vi "Trajectory Builder.vi"() -> ()   [LabVIEW 2025]
uses:
  Types/Limits.ctl
  Types/Overrides.ctl
  Types/Trajectory Data.ctl
  Types/Segment Type.ctl
  Types/Path Type.ctl
  Types/Drive Type.ctl
  Types/Angluar Limits.ctl
  Types/Command Editor Info.ctl
  Types/Single Cmd Info.ctl
  <vilib>/picture/picture.llb/imagedata.ctl
  <vilib>/Utility/miscctls.llb/LVPositionTypeDef.ctl
  <vilib>/Utility/miscctls.llb/LVRowAndColumnTypeDef.ctl
  Types/Internal Path Stuff.ctl
  <vilib>/event_ctls.llb/lveventtype.ctl
  6a65ebb4-e776-4ba2-b94f-6ff829af6114.vi
  6a65ebb4-e776-4ba2-b94f-6ff829af6114.vi/c0db33a9-eb6c-44d9-b982-8563e05d2734.vi
  6a65ebb4-e776-4ba2-b94f-6ff829af6114.vi/ae3535a8-0066-4e8d-a5de-b07ac05a7c65.vi
  6a65ebb4-e776-4ba2-b94f-6ff829af6114.vi/dda8e586-731b-4197-ad83-6a4d05585a0a.vi
  Global Settings.vi
  <vilib>/Utility/cursorutil.llb/Set Cursor (Icon Pict).vi
  <vilib>/Comparison/Less/Less Functor/Less Functor.lvclass
panel:
  in  "Correct at Beginning \nof Path":bool
  in  "Zero Translational\n Velocity":bool
  in  "Pickup Balls":bool
  in  "Delete":bool
  out "Picture":picture
  in  "New Page Selector":T1(radio)
  in  "Push":bool
  out "?":bool
  out "RS":bool=TRUE
  in  "Cache":T5
  in  "Zero Velocity":bool
  in  "Reverse Path":bool
  in  "Robot Backwards":bool
  out "Duration (s)":dbl format="%#.4g"
  out "Distance (ft)":dbl format="%#.1g"
  in  "Instructions":string="Directions:\nUse mouse to ...\n    move robot position (rectangle with arrow)\n    rotate robot (red arrow)\n    move waypoints (numbered circles)\nClick in open space to add a waypoint\nShift click to delete a waypoint\nHover over a waypoint and use arrow keys to nudge\n\nTime slider and Play button will run robot along path to test for collisions.\n\nNew creates a new path at default location\n\nAppend creates a path using current path's position and heading.\n\nTo add a command, move robot using Time slider and double click the Command in Palette.\n\nYou can modify command timing in the graph or Command Sequencer tree.\n\nEnable/disable a command by clicking on the enable column item.\n\nDelete a command by shift-clicking in the enable column.\n\nTo configure command parameters, Select the command name in the tree, Open Panel, enter parameters, and Inhale the parameters.\n\nYou may sometimes want to type values into WayPoints directly.\n\nOverrides allow you to set accel and V limits for any turn."
  out "Command Palette":picture
  in  "Directory":bool
  in  "Tab Control":T1(tab)
  in  "Vertical Reflection":bool
  in  "Angular Limits":T6={"Velocity (deg/s)"=6.0, "Accel (deg/s^2)"=360.0, "Jerk (deg/s^3)"=1000.0} {"Jerk (deg/s^3)" min=0.01 step=1.0; "Accel (deg/s^2)" min=0.01; "Velocity (deg/s)" min=0.01}
  in  "Path Type":T7
  in  "Overrides":T8=[{"Count"="1", "Angular Override"=0.0, "Enabled?"=FALSE, "Velocity Override"=6.0, "Angle Override"=nan}] {"Angle Override" step=5.0; "Velocity Override" step=5.0; "Angular Override" step=5.0}
  in  "Horizontal Reflection":bool
  in  "Sample Period (s)":dbl=0.02 min=0.001 max=1.0 format="%#_6p"
  in  "Limits":T9={"Velocity (fps)"=6.0, "Accel (fps^2)"=15.0, "Jerk (fps^3)"=150.0, "StoopidFast (fps)"=6.0} {"StoopidFast (fps)" min=0.01; "Jerk (fps^3)" min=0.01 step=1.0; "Accel (fps^2)" min=0.01; "Velocity (fps)" min=0.01}
  in  "Conditions":T10 {"vFinal (fps)" min=0.0; "vInitial (fps)" min=0.0}
  in  "Drive Type":T11=enum."Holonomic"
  in  "Turn Rate (Bezier)":dbl=5.0 format="%#_13g"
  in  "Origin Reflection":bool
  in  "Current Limit":dbl=50.0 min=0.01
  in  "WayPoints":cluster{"x":dbl, "y":dbl, "th":dbl}[](array[cluster])
  in  "Turn Angle Limit (deg)":dbl=90.0
  in  "Allow Angles > 90":bool=TRUE
  in  "Stoopid Overlap %":dbl min=0.0
  in  "Unjank":bool
  in  "Turn Deceleration":bool=TRUE
  in  "Turn Acceleration":bool=TRUE
  out "Trajectory Data":T12
  in  "Open Command":bool
  in  "Inhale":bool
  in  "Command Sequence":string(tree)
  in  "Projects":u16(ring) items=["Rebuilt 2468.lvproj"]
  in  "Refresh":bool
  in  "Snap to foot":bool
  in  "Angle Limiter":enum16{"90", "45", "15", "1"}(ring)=enum."15"
  in  "Snap robot to baseline":bool
  in  "Background":u16(ring) items=["Rebuilt", "Reefscape"]
  in  "Robot Color":u32(colorbox)=14421504
  out "Field Size (ft)":cluster{"width":dbl, "height":dbl}={"width"=26.4166, "height"=57.5729} {"width" format="%#.2g"; "height" format="%#.2g"}
  in  "Robot Size (in)":cluster{"width":dbl, "height":dbl}={"width"=24.0, "height"=30.0}
  in  "Hide Path":bool
  in  "Time (s)":dbl(slide) scale=0.0..1.6400000000000001 scale format="%#.1g"
  in  "Play":bool
  out "fps":dbl[](graph)
  in  "Append":bool
  in  "Open":i32[](listbox)
  in  "Filename":string
  in  "Save":bool
  in  "New":bool
  # "Command Palette"
  # "StupidFast makes each linear segment into a\nvelocity ramp to max speed (for clothoid paths only)"
  # "Nicotine"
  # "A"
  # "V"
  # "O"
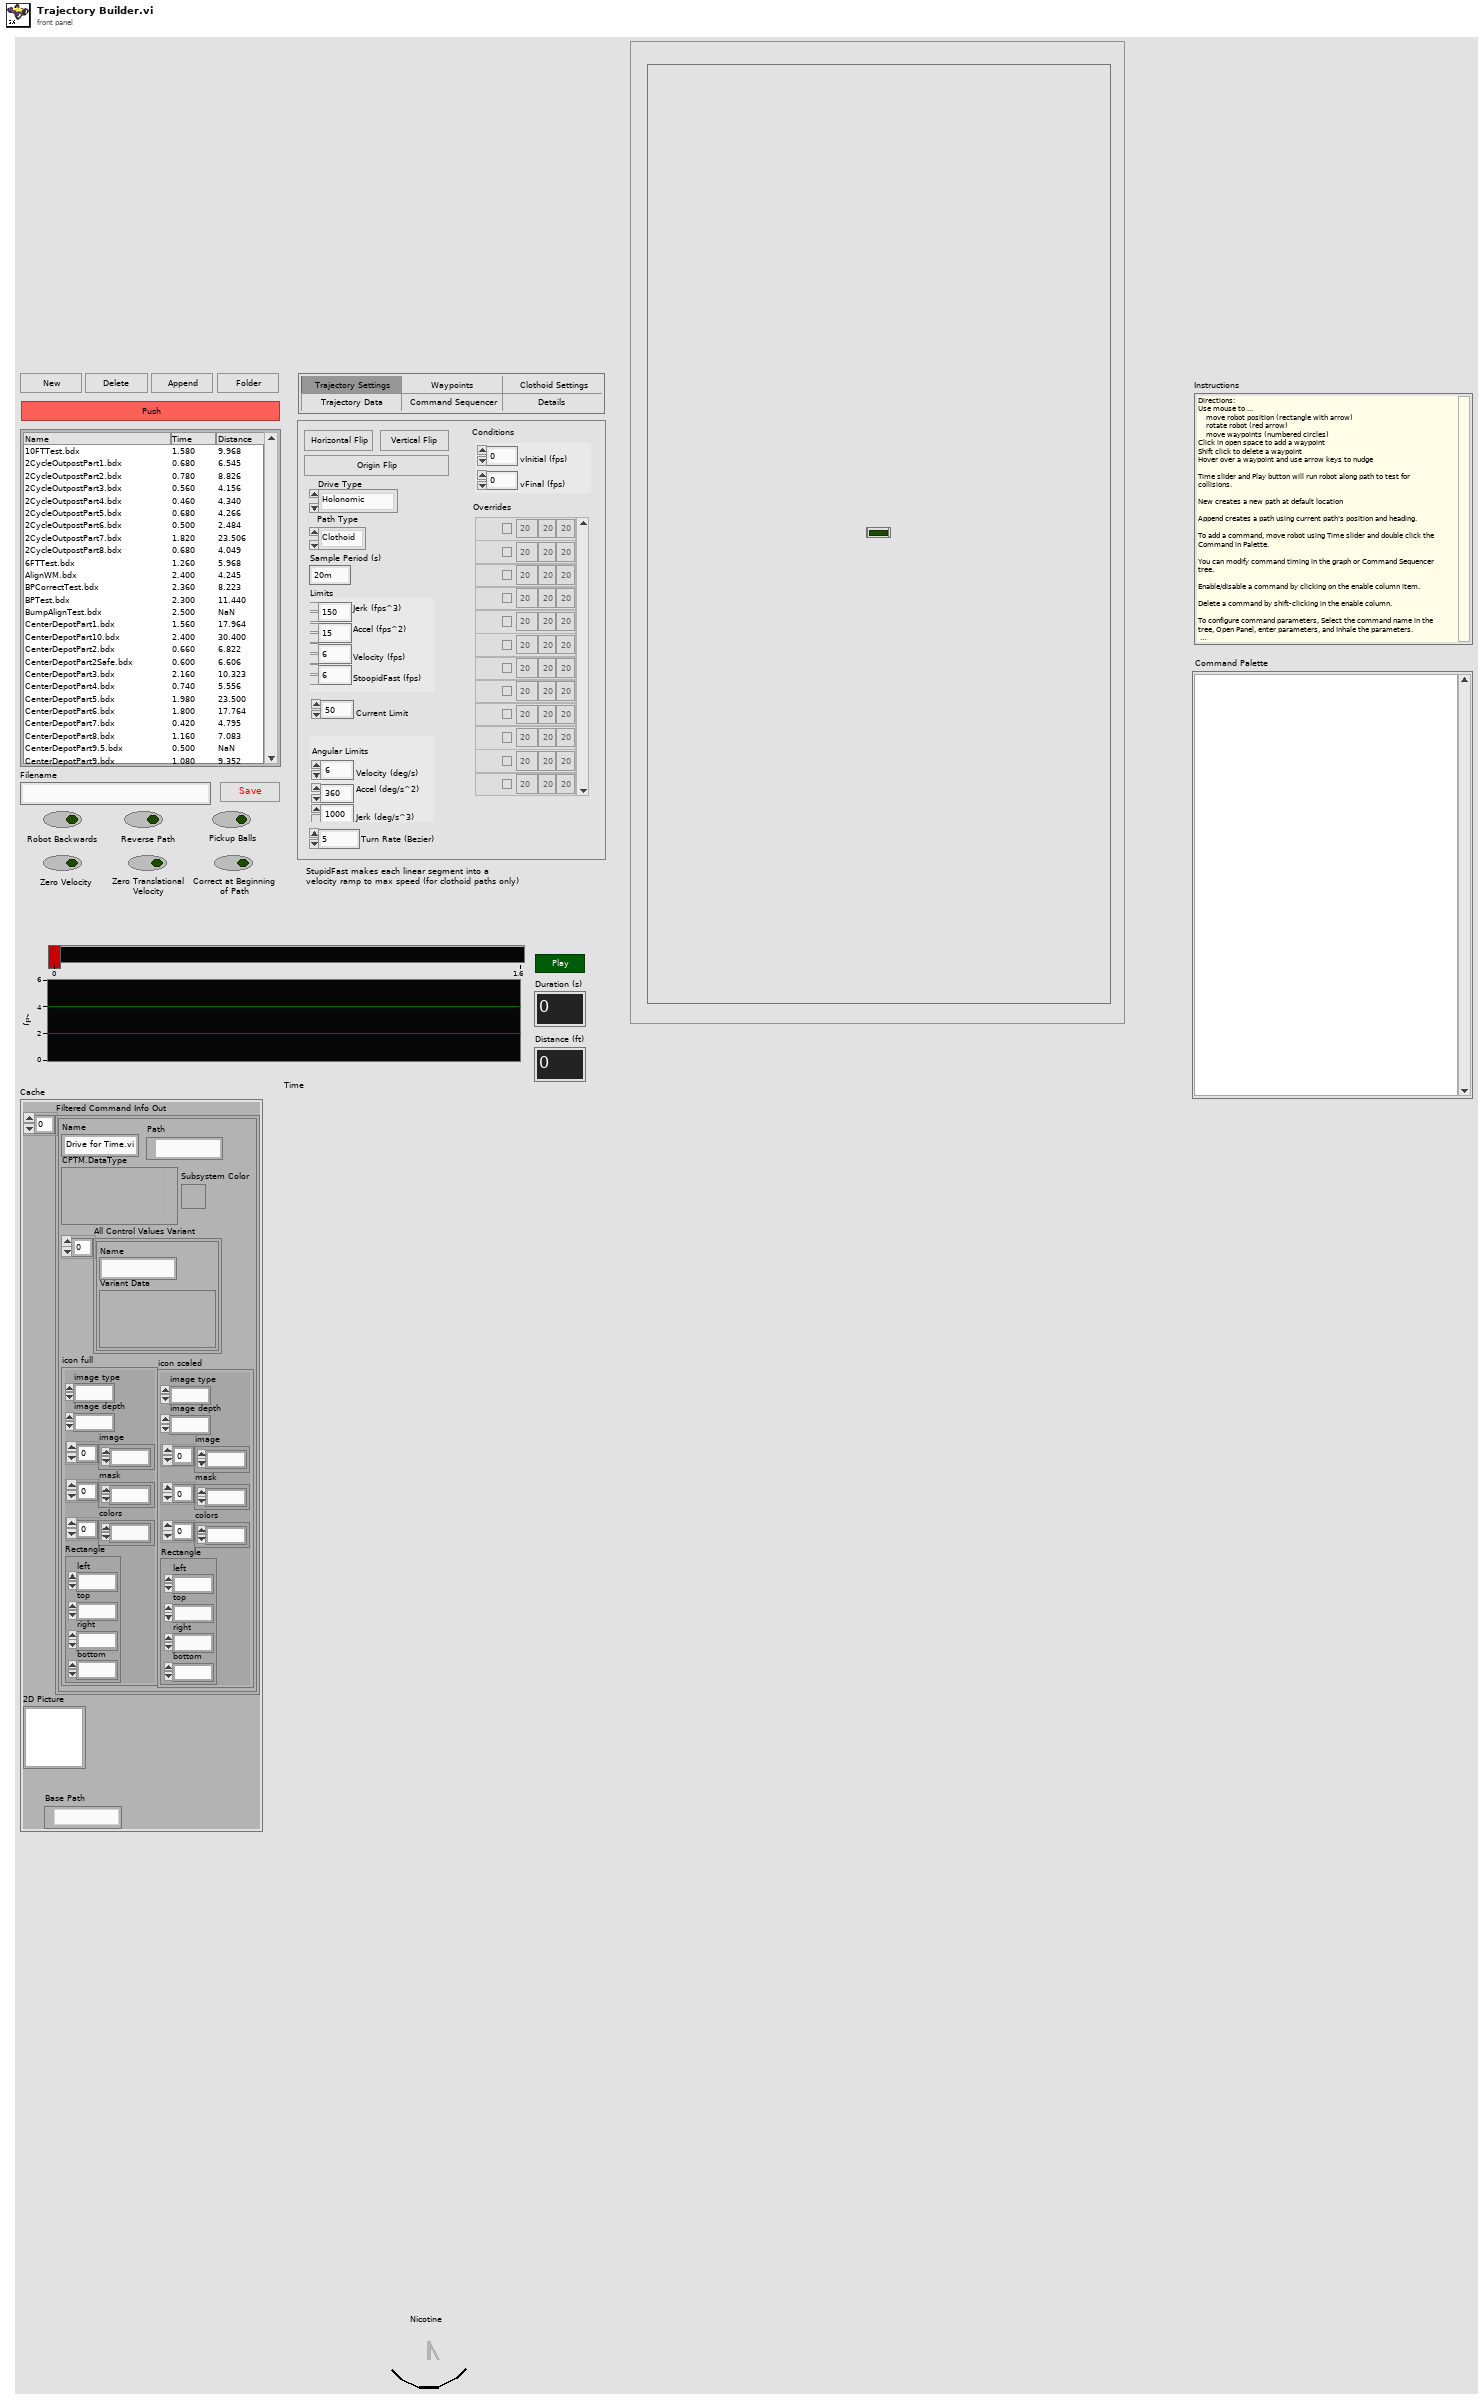
[diagram p1: front panel]
types:
  T1 = enum32{"Trajectory Settings", "Waypoints", "Clothoid Settings", "Trajectory Data", "Command Sequencer", "Details"}
  T2 = typedef "Command Editor Info.ctl" = T3[]
  T3 = typedef "Single Cmd Info.ctl" = cluster{"Name":string, "CPTM.DataType":variant, "All Control Values Variant":cluster{"Name":string, "Variant Data":variant}[], "icon full":T4, "icon scaled":T4, "Path":path, "Subsystem Color":u32}
  T4 = typedef "imagedata.ctl" = cluster{"image type":i32, "image depth":i32, "image":u8[], "mask":u8[], "colors":u32[], "Rectangle":cluster{"left":i16, "top":i16, "right":i16, "bottom":i16}}
  T5 = cluster{"Filtered Command Info Out":T2, "2D Picture":picture, "Base Path":path}
  T6 = typedef "Angluar Limits.ctl" = cluster{"Velocity (deg/s)":dbl, "Accel (deg/s^2)":dbl, "Jerk (deg/s^3)":dbl}
  T7 = typedef "Path Type.ctl" = enum16{"Clothoid", "Bezier"}
  T8 = typedef "Overrides.ctl" = cluster{"Count":string, "Angular Override":dbl, "Enabled?":bool, "Velocity Override":dbl, "Angle Override":dbl}[]
  T9 = typedef "Limits.ctl" = cluster{"Velocity (fps)":dbl, "Accel (fps^2)":dbl, "Jerk (fps^3)":dbl, "StoopidFast (fps)":dbl}
  T10 = cluster{"vInitial (fps)":dbl, "vFinal (fps)":dbl}
  T11 = typedef "Drive Type.ctl" = enum16{"Nonholonomic", "Holonomic"}
  T12 = typedef "Trajectory Data.ctl" = cluster{"Segment Name":string, "Type":T13, "Traj Pos Points":cluster{"x":dbl, "y":dbl, "th":dbl}[], "Traj Vel Points":cluster{"V":dbl, "Omega":dbl, "V vector":cluster{"y":dbl, "x":dbl}}[], "Accel Index":i32, "Decel Index":i32}[]
  T13 = typedef "Segment Type.ctl" = enum16{"Accel Straight", "Const Straight", "Blend", "Circle", "Bezier"}
  T14 = cluster{"Sample Period (s)":dbl, "Limits":T9, "Conditions":cluster{"vInitial (fps)":dbl, "vFinal (fps)":dbl}, "Overrides":T8, "Angular Limits":T6}
  T15 = typedef "LVRowAndColumnTypeDef.ctl" = cluster{"Row":i32, "Column":i32}
  T16 = typedef "LVPositionTypeDef.ctl" = cluster{"Left":i32, "Top":i32}
  T17 = cluster{"Index":i32, "Pt Test Results":enum16{"Miss", "Rect Hit", "Arrow Hit"}}
  T18 = cluster{"Drag Object":cluster{"Index":i32, "x":dbl, "y":dbl}, "Hover Object":cluster{"Index":i32, "Pt Test Results":enum16{"Miss", "Rect Hit", "Arrow Hit"}}, "Filename":string}
  T19 = cluster{"Trajectory Data":T12, "Points":cluster{"x":dbl, "y":dbl, "th":dbl}[], "output cluster":cluster{"Sample Period (s)":dbl, "Limits":T9, "Conditions":cluster{"vInitial (fps)":dbl, "vFinal (fps)":dbl}, "Overrides":T8, "Angular Limits":T6}, cluster{"Time (s)":dbl, T3, bool}[]}
  T20 = typedef "Internal Path Stuff.ctl" = cluster{"Trajectory Data":T12, "Updated Waypoints":cluster{"x":dbl, "y":dbl, "th":dbl}[], cluster{"Sample Period (s)":dbl, "Limits":T9, "Conditions":cluster{"vInitial (fps)":dbl, "vFinal (fps)":dbl}, "Overrides":T8, "Angular Limits":T6}, "Commands out":cluster{"Time (s)":dbl, T3, bool}[]}
  T21 = typedef "lveventtype.ctl" = enum32{"Null", "Timeout", "Annotation Menu Selection", "Annotation Menu Selection?", "App Instance Close", "App Instance Close?", "Autoscale Range Change", "Bookmark Info Change", "Cell Edit", "Cell Edit?", "Cursor Grab", "Cursor Grab?", "Cursor Menu Selection", "Cursor Menu Selection?", "Cursor Move", "Cursor Release", "Data Change", "Direction Change", "Display State Change", "Drag Ended", "Drag Enter", "Drag Leave", "Drag Over", "Drag Source Update", "Drag Starting", "Drag Starting?", "Drop", "Exec State Change", "Key Down", "Key Down?", "Key Repeat", "Key Repeat?", "Key Up", "Listbox Double Click", "Menu Activation?", "Menu Selection (App)", "Menu Selection? (App)", "Menu Selection (User)", "Mouse Down", "Mouse Down?", "Mouse Enter", "Mouse Leave", "Mouse Move", "Mouse Up", "Mouse Wheel", "NI Security User Change (App)", "Pane Size", "Panel Close", "Panel Close?", "Panel Resize", "Plot Attribute Change", "Scale Range Change", "Shortcut Menu Activation?", "Shortcut Menu Selection (App)", "Shortcut Menu Selection? (App)", "Shortcut Menu Selection (User)", "Tree Double Click", "Tree Drag", "Tree Drag?", "Tree Drop", "Tree Drop?", "Tree Item Close", "Tree Item Close?", "Tree Item Open", "Tree Item Open?", "User Event", "Value Change"}
  T22 = enum32{"Invalid", "Standard", "Closed", "Hidden", "Minimized", "Maximized"}
  T23 = cluster{"width":dbl, "height":dbl, "width":dbl, "height":dbl}
  T24 = cluster{"status":bool, "code":bool, "source":bool}
  T25 = cluster{"Robot Backwards":bool, "Reverse Path":bool}
  T26 = cluster{cluster{"Robot Backwards":bool, "Reverse Path":bool}, "Trajectory Data":T12, "sorted array out":cluster{"Time (s)":dbl, T3, bool}[], cluster{"Sample Period (s)":dbl, "Limits":T9, "Conditions":cluster{"vInitial (fps)":dbl, "vFinal (fps)":dbl}, "Overrides":T8, "Angular Limits":T6}, "Updated Waypoints":cluster{"x":dbl, "y":dbl, "th":dbl}[], cluster{"Time (s)":dbl, "Distance (ft)":dbl}, "Zero Velocity":bool, cluster{"Drive Type":T11, "Path Type":T7}, "Pickup Balls":bool, "Current Limit":dbl, "Zero Translational\n Velocity":bool, "Correct at Beginning \nof Path":bool}
  T27 = cluster{"Trajectory Data":T12, "Updated Waypoints":cluster{"x":dbl, "y":dbl, "th":dbl}[], cluster{"Sample Period (s)":dbl, "Limits":T9, "Conditions":cluster{"vInitial (fps)":dbl, "vFinal (fps)":dbl}, "Overrides":T8, "Angular Limits":T6}, "sorted array out":cluster{"Time (s)":dbl, T3, bool}[]}
  T28 = cluster{"Sample Period (s)":dbl, cluster{"Velocity (fps)":dbl, "Accel (fps^2)":dbl, "Jerk (fps^3)":dbl, "StoopidFast (fps)":dbl}, "Conditions":cluster{"vInitial (fps)":dbl, "vFinal (fps)":dbl}, "Overrides":T8, "Angular Limits":T6}
  T29 = cluster{"Velocity (fps)":dbl, "Accel (fps^2)":dbl, "Jerk (fps^3)":dbl, "StoopidFast (fps)":dbl}
  T30 = cluster{"Trajectory Data":T12, "Points out":cluster{"x":dbl, "y":dbl, "th":dbl}[], "Fields":cluster{"Sample Period (s)":dbl, cluster{"Velocity (fps)":dbl, "Accel (fps^2)":dbl, "Jerk (fps^3)":dbl, "StoopidFast (fps)":dbl}, "Conditions":cluster{"vInitial (fps)":dbl, "vFinal (fps)":dbl}, "Overrides":T8, "Angular Limits":T6}, "Commands out":cluster{"Time (s)":dbl, T3, bool}[]}
  T31 = typedef "LVPoint32TypeDef.ctl" = cluster{"Horizontal":i32, "Vertical":i32}
  T32 = cluster{"Shift":bool, "Ctrl":bool, "Alt":bool, "Cmd":bool, "Opt":bool}
  T33 = typedef "LVBoundsTypeDef.ctl" = cluster{"Width":u32, "Height":u32}
  T34 = cluster{"Snap robot to baseline":bool, "Snap to foot":bool, "Angle Limiter":enum16{"90", "45", "15", "1"}}
  T35 = cluster{i32, "Pt Test Results":enum16{"Miss", "Rect Hit", "Arrow Hit"}}
  T36 = typedef "eventvkey.ctl" = enum16{"ASCII", "Enter", "Return", "Shift", "Ctrl", "Alt", "Cmd", "Opt", "Caps", "NumLock", "Clear", "Break", "Up", "Down", "Left", "Right", "Insert", "Delete", "Home", "End", "PageUp", "PageDown", "Escape", "Help", "Pause", "ScrollLock", "F1", "F2", "F3", "F4", "F5", "F6", "F7", "F8", "F9", "F10", "F11", "F12", "F13", "F14", "F15", "F16", "F17", "F18", "F19", "F20", "F21", "F22", "F23", "F24", "Play", "VolumeUp", "VolumeDown", "Mute", "Two Byte Char"}
  T37 = cluster{"Name":string, "CPTM.DataType":variant, "Get All Control Values Variant":cluster{"Name":string, "Variant Data":variant}[], "Color 256":T4, "Subsystem Color":u32}[]
  T38 = cluster{"Filtered Command Info Out":T2, "2D Picture":picture, "stripped path":path}
  T39 = cluster{"Horizontal":dbl, "Vertical":dbl, "th":dbl}
  T40 = cluster{"Name":string, "Color":u32, "Style":i32, "Point Style":i32, "Name Visible":bool, "Allow Drag":bool, "Annotation Mode":i32, "Plot":i32, "Index":i32, "Position":cluster{"X":dbl, "Y":dbl}, "X Scale":i32, "Y Scale":u32, "Show Arrow":bool, "Lock Name":bool, "Plot Area":i32, "Label Offset":cluster{"X":dbl, "Y":dbl}}[]
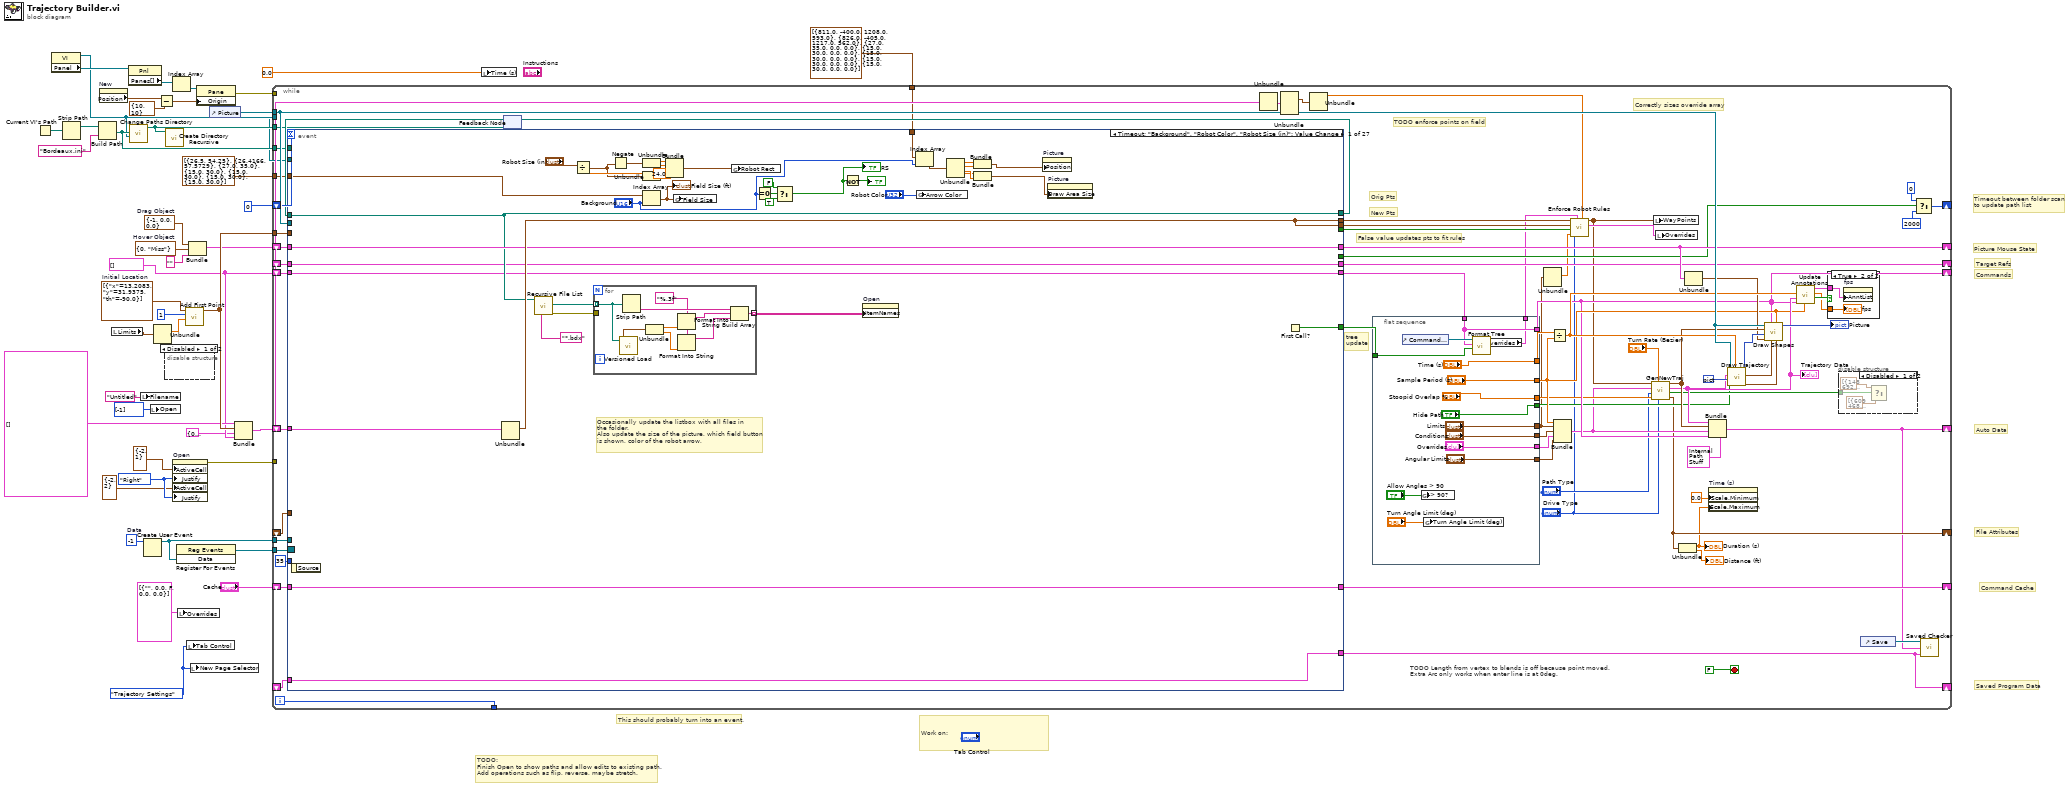
[diagram p0: block diagram]
diagram:
  w3 = T1."Trajectory Settings" ("Tab Control")
  w12 = enum16{"Left", "Center", "Right"}."Right" ("Active Cell:Cell Justification")
  w19 = cluster{"Time (s)":dbl, T3, bool}[] []
  w33 = -1  # Data
  w30 = T17 {"Index"=0, "Pt Test Results"=enum."Miss"}  # Hover Object
  w29 = cluster{"Index":i32, "x":dbl, "y":dbl} {"Index"=-1, "x"=0.0, "y"=0.0}  # Drag Object
  w41 = cluster{"x":dbl, "y":dbl, "th":dbl}[] [{"x"=13.2083, "y"=31.9375, "th"=-90.0}]  # Initial Location
  # "Saved Program Data"
  # "Command Cache"
  # "File Attributes"
  # "Commands"
  # "Target Refs"
  # "Picture Mouse State"
  # "Auto Data"
  # "Timeout between folder scan\nto update path list"
  # "This should probably turn into an event."
  # "Work on:"
  # "TODO: \nFinish Open to show paths and allow edits to existing path.\nAdd operations such as flip, reverse, maybe stretch."
  n1 = Current VI's Path() -> (path=w17:path)
  n2 = property class="VI"() -> (reference out=w8:refnum<vi>, "Panel"=w27:refnum<vi>)  [unwired: 2 in, 1 out]
  n3 = Strip Path(path=w17) -> (stripped path=w16:path)  [unwired: 1 out]
  n4 = Build Path(base path=w16, name or relative path="Bordeaux.ini" ("format string")) -> (appended path=w10:path)
  n5 = property on="New" class="Bool"() -> ("Position"=w23:T16)  [unwired: 2 in, 2 out]
  n6 = local read "Limits"() -> (w38:T9)
  n7 = property class="Pnl"(reference=w27) -> ("Panes[]"=w26:refnum<vi>[])  [unwired: 1 in, 2 out]
  n8 = call "Change Paths Directory.vi"("VI Refnum"=w8, "config path"=w10) -> ("Bordeaux paths out"=w9:path)  [unwired: 9 in]
  n9 = local write "Filename"("Untitled" ("Filename")) -> ()
  n10 = Create User Event(user event datatype=w33) -> (user event=w34:refnum<user-event>)  [unwired: 1 in, 1 out]
  n11 = local write "Open"(i32[] [-1] ("Open")) -> ()
  n12 = Unbundle(w38) -> ("Accel (fps^2)"=w37:dbl)  [unwired: 3 out]
  n13 = Subtract(x=w23, y=T16 {"Left"=10, "Top"=10}) -> (x-y=w22:T16)
  n14 = disable-structure shown="Disabled" {
    frame Disabled {
    }
    frame Enabled {
    }
  }
  n15 = call <vilib>:"Create Directory Recursive.vi"("directory"=w9) -> ()  [unwired: 4 in, 3 out]
  n16 = Index Array(array=w26) -> (element=w25:refnum<vi>)  [unwired: 1 in]
  n17 = property on="Open" class="MCListbox (strict)"("ActiveCell"=T15 {"Row"=-2, "Column"=1} ("Active Cell:Active Cell"), "Justify"=w12, "ActiveCell"=T15 {"Row"=-2, "Column"=2} ("Active Cell:Active Cell"), "Justify"=w12) -> (error out=w13:errorcluster)  [unwired: 2 in, 1 out]
  n18 = register-events(w34) -> (reference out=w35:refnum<event-registration>)  [unwired: 2 in, 1 out]
  n19 = local write "Overrides"(T8 [{"Count"="", "Angular Override"=0.0, "Enabled?"=FALSE, "Velocity Override"=0.0, "Angle Override"=0.0}] ("Overrides")) -> ()
  n20 = call "Add First Point.vi"("Accel (f/s^2)"=w37, "Time (s)"=1 ("th"), "Initial Points"=w41) -> ("Points"=w32:cluster{"x":dbl, "y":dbl, "th":dbl}[])  [unwired: 8 in]
  n21 = local write "Tab Control"(w3) -> ()
  n22 = Bundle("Drag Object"=w29, "Hover Object"=w30, "Filename"="") -> (w28:T18)  [unwired: 1 in]
  n23 = local write "New Page Selector"(w3) -> ()
  n24 = property class="Pane"(reference=w25, "Origin"=w22) -> (error out=w21:errorcluster)  [unwired: 1 in, 1 out]
  n25 = control-ref of="Picture"() -> (w43:refnum<vi>)
  n26 = Bundle("Trajectory Data"=T12 [], "Points"=w32, "output cluster"=T14 {"Sample Period (s)"=0.2, "Limits"={"Velocity (fps)"=6.0, "Accel (fps^2)"=32.0, "Jerk (fps^3)"=1500.0, "StoopidFast (fps)"=12.0}, "Conditions"={"vInitial (fps)"=0.0, "vFinal (fps)"=0.0}, "Overrides"=[], "Angular Limits"={"Velocity (deg/s)"=0.0, "Accel (deg/s^2)"=0.0, "Jerk (deg/s^3)"=0.0}}, w19) -> (w6:T19)  [unwired: 1 in]
  n27 = while {
    tunnel: w32 -> [w117]
    tunnel: w43 -> [w116]
    shift-right: [w89] -> _
    shift-left: 0 -> [w110]
    shift-right: [w58] -> _
    shift-left: _ -> [w109]
    tunnel: w9 -> [w96]
    tunnel: w35 -> [w104]
    tunnel: w34 -> [w103]
    shift-right: [w101] -> _
    shift-left: _ -> [w102]
    shift-right: [w53] -> _
    shift-left: w6 -> [w73]
    shift-right: [w93] -> _
    shift-left: w28 -> [w94]
    shift-right: [w85] -> _
    shift-left: _ -> [w84]
    shift-right: [w82] -> _
    shift-left: "Cache" -> [w83]
    shift-right: [w75] -> _
    shift-left: w19 -> [w80]
    tunnel: w21 -> [_]
    tunnel: cluster{"width":dbl, "height":dbl}[] [{"width"=26.5, "height"=54.25}, {"width"=26.4166, "height"=57.5729}, {"width"=27.0, "height"=35.0}, {"width"=15.0, "height"=30.0}, {"width"=15.0, "height"=30.0}, {"width"=15.0, "height"=30.0}, {"width"=15.0, "height"=30.0}] -> [w70]
    tunnel: [w67] -> _
    tunnel: w13 -> [_]
    tunnel: w10 -> [w61]
    tunnel: w8 -> [w60]
    tunnel: cluster{"width":dbl, "height":dbl, dbl, dbl}[] [{"width"=811.0, "height"=-400.0, 1208.0, 593.0}, {"width"=826.0, "height"=-405.0, 1217.0, 562.0}, {"width"=27.0, "height"=35.0, 0.0, 0.0}, {"width"=15.0, "height"=30.0, 0.0, 0.0}, {"width"=15.0, "height"=30.0, 0.0, 0.0}, {"width"=15.0, "height"=30.0, 0.0, 0.0}, {"width"=15.0, "height"=30.0, 0.0, 0.0}] -> [w44]
    i -> [w67]
    stop <- FALSE stop-if-true
    # "False value updates pts to fit rules"
    # "tree\nupdate"
    # "New Pts"
    # "Orig Pts"
    # "Correctly sizes override array"
    # "TODO Length from vertex to blends is off because point moved.\nExtra Arc only works when enter line is at 0deg."
    # "TODO enforce points on field"
    n28 = feedback #1(w96) -> (w97:path)
    n29 = event shown="[0] Timeout;  \"Background\", \"Robot Color\", \"Robot Size (in)\": Value Change" {
      selector: w104 -> [_ _ _ _ _ _ _ _ _ _ _ _ _ _ _ _ _ _ _ _ _ _ _ _ _ _ _]
      dyn-events: _ -> [_ _ _ _ _ _ _ _ _ _ _ _ _ _ _ _ _ _ _ _ _ _ _ _ _ _ _]
      timeout: w110 -> [_ _ _ _ _ _ _ _ _ _ _ _ _ _ _ _ _ _ _ _ _ _ _ _ _ _ _]
      tunnel: [w169 w208 w241 w281 w300 w330 w371 w386 w398 w414 w473 w505 w620 w662 w767 w794 w820 w836 w858 w877 w918 w967 w1001 w1050 w1077 w1109 w1140] -> w108
      tunnel: w117 -> [_ _ w241 _ _ _ _ _ w398 w415 _ _ _ _ _ _ _ _ _ _ _ _ _ _ _ _ _]
      tunnel: w116 -> [_ _ _ _ _ _ _ _ _ _ _ w504 w606 _ w754 _ _ _ _ _ _ _ _ _ _ _ _]
      tunnel: w97 -> [w167 w206 w249 w270 w305 w327 w363 w382 w395 w419 w472 w502 w617 w676 w768 w808 w823 w838 w864 w881 w922 w973 w1006 w1054 w1082 w1114 w1145]
      tunnel: [w169 w208 w246 w281 w300 w330 w371 w386 w396 w417 w473 w499 w614 w654 w752 w794 w820 w836 w858 w877 w918 w967 w1001 w1050 w1077 w1109 w1140] -> w107
      tunnel: w109 -> [_ _ _ _ _ w322 _ _ _ _ _ _ _ _ _ _ _ _ _ _ _ _ _ _ _ _ _]
      tunnel: [_ _ w240 TRUE ("Flip Over Center") _ _ _ _ _ TRUE ("Flip Over Center") _ _ _ TRUE ("Flip Over Center") _ _ _ _ _ _ _ _ _ _ _ _ _] -> w59
      tunnel: [w167 w206 w249 w270 w305 w327 w363 w375 w395 w419 w472 w502 w617 w676 w768 w808 w823 w838 w864 w881 w922 w973 w1006 w1054 w1082 w1114 w1145] -> w98
      tunnel: w103 -> [_ _ _ _ w304 _ _ _ _ _ _ _ _ _ _ w789 _ _ _ _ _ _ _ _ _ _ _]
      tunnel: [w171 w213 w248 w271 w303 w339 w373 w388 w403 w424 w480 w501 w616 w675 w755 w806 w822 w839 w863 w880 w921 w972 w1005 w1053 w1081 w1113 w1144] -> w101
      tunnel: w102 -> [w171 w213 w248 w271 w303 _ w373 w388 w403 w424 _ w501 w616 w675 w755 w806 w822 w839 w863 w880 w921 w972 w1005 w1053 w1081 w1113 w1144]
      tunnel: w73 -> [w170 w209 w247 w269 w301 w338 w372 w387 w397 w418 _ w500 w615 w674 w753 w795 w821 w837 _ w878 w919 w969 w1002 w1051 w1078 w1110 w1141]
      tunnel: w94 -> [w168 w212 w245 w268 w299 w337 w368 w389 w402 w423 w488 w496 w607 w673 w750 w793 w819 w835 w862 w876 w917 w971 w1004 w1036 w1080 w1112 w1143]
      tunnel: [w168 w212 w245 w268 w299 w337 w369 w389 w402 w423 w488 w498 w611 w673 w750 w793 w819 w835 w862 w876 w917 w971 w1004 w1037 w1080 w1112 w1143] -> w93
      tunnel: [_ _ _ _ _ TRUE _ TRUE _ _ _ _ _ _ _ _ _ _ _ _ _ _ _ _ _ _ _] -> w88
      tunnel: [w166 w207 w243 w267 w298 w335 w362 w380 w401 w422 w487 w492 w609 w672 w748 w792 w814 w832 w861 w879 w920 w970 w1003 w1052 w1079 w1111 w1142] -> w85
      tunnel: w84 -> [w166 w207 w243 w267 w298 w335 w362 w380 w401 w422 w487 w492 w609 w672 w748 w792 w817 w832 w861 w879 w920 w970 w1003 w1052 w1079 w1111 w1142]
      tunnel: w83 -> [w165 w211 w244 w266 w297 w334 w361 w379 w400 w421 w486 w494 w608 w671 w747 w791 w816 _ w860 w865 w910 w960 w986 w1034 w1063 w1100 w1128]
      tunnel: [w165 w211 w244 w266 w297 w334 w361 w379 w400 w421 w486 w494 w608 w671 w747 w791 w816 w834 w860 w865 w910 w960 w986 w1034 w1063 w1100 w1128] -> w82
      tunnel: 35 -> [_ _ _ _ _ _ _ _ _ _ _ _ _ _ _ _ _ _ _ _ _ _ _ _ _ w1102 w1136]
      tunnel: w80 -> [w164 w210 _ w265 w296 w316 w370 w377 w399 w416 _ w493 w605 w670 w746 w790 w815 w833 w859 w866 w908 w965 w989 w1039 w1066 w1101 w1130]
      tunnel: [w164 w210 _ w265 w296 w316 w370 w377 w399 w416 w484 w493 w605 w670 w746 w790 w815 w833 w859 w866 w912 w966 w987 w1039 w1061 w1101 w1127] -> w79
      tunnel: [w163 _ w240 TRUE ("First Call?: T/F") _ _ _ _ _ TRUE ("First Call?: T/F") TRUE _ _ _ _ _ _ _ _ w869 w911 TRUE w988 _ w1065 _ TRUE] -> w78
      tunnel: w70 -> [w152 _ _ _ _ _ _ _ _ _ _ _ w595 w661 w739 _ _ _ _ _ _ _ _ _ _ _ _]
      tunnel: w61 -> [_ _ _ _ _ _ _ w376 _ _ _ _ _ _ _ _ _ _ _ _ _ _ _ _ _ _ _]
      tunnel: w60 -> [_ _ _ _ _ _ _ w374 _ _ _ _ _ _ _ _ _ _ _ _ _ _ _ _ _ _ _]
      tunnel: w44 -> [w143 _ _ _ _ _ _ _ _ _ _ _ _ _ _ _ _ _ _ _ _ _ _ _ _ _ _]
      event Timeout; "Background", "Robot Color", "Robot Size (in)": Value Change {
        # "Occasionally update the listbox with all files in\nthe folder.\nAlso update the size of the picture, which field button\nis shown, color of the robot arrow,"
        n30 = event-data() -> ()  [unwired: 1 in, 1 out]
        n31 = Unbundle(w170) -> ("Updated Waypoints"=w169:cluster{"x":dbl, "y":dbl, "th":dbl}[])  [unwired: 3 out]
        n32 = call <vilib>:"Recursive File List.vi"("pattern"="*.bdx", "Folder Path"=w167) -> ("error out"=w172:errorcluster, "All Files in Dir"=w174:path[])  [unwired: 5 in, 3 out]
        n33 = Divide(x="Robot Size (in)", y=24.0 ("width")) -> (x/y=w159:cluster{"width":dbl, "height":dbl})
        n34 = for {
          tunnel: w174 -> [w181] mode=indexing
          tunnel: [w183] -> w173 mode=indexing
          tunnel: w172 -> [_]
          w175 = "%.3f" ("format string")
          n35 = call "Versioned Load.vi"("path"=w181) -> ("Overall"=w180:cluster{"Time (s)":dbl, "Distance (ft)":dbl})  [unwired: 15 in, 11 out]
          n36 = Strip Path(path=w181) -> (name=w182:string)  [unwired: 1 out]
          n37 = Unbundle(w180) -> ("Time (s)"=w179:dbl, "Distance (ft)"=w178:dbl)
          n38 = Format Into String(format string=w175, w179) -> (resulting string=w177:string)  [unwired: 2 in, 1 out]
          n39 = Format Into String(format string=w175, w178) -> (resulting string=w176:string)  [unwired: 2 in, 1 out]
          n40 = Build Array(w182, w177, w176) -> (w183:string[])
        }
        n41 = Negate(x=w159) -> (-x=w160:cluster{"width":dbl, "height":dbl})
        n42 = Unbundle(w160) -> ("width"=w158:dbl, "height"=w157:dbl)
        n43 = Unbundle(w159) -> ("width"=w156:dbl, "height"=w155:dbl)
        n44 = Index Array(array=w152, index="Background") -> (element=w151:cluster{"width":dbl, "height":dbl})
        "Field Size (ft)" <- w151
        n45 = Bundle("width"=w158, "height"=w157, "width"=w156, "height"=w155) -> (w154:T23)  [unwired: 1 in]
        n46 = global write "Global Settings.vi" "Field Size"(w151) -> ()
        n47 = global write "Global Settings.vi" "Robot Rect"(w154) -> ()
        n48 = Equal To 0?(x="Background") -> (x = 0?=w149:bool)
        n49 = Select(t=FALSE, s=w149, f=TRUE) -> (s? t:f=w147:bool)
        "RS" <- w147
        n50 = Not(x=w147) -> (.not. x?=→"?":bool)
        n51 = property on="Open" class="MCListbox (strict)"("ItemNames"=w173) -> ()  [unwired: 2 in, 2 out]
        n52 = Index Array(array=w143, index="Background") -> (element=w142:cluster{"width":dbl, "height":dbl, dbl, dbl})
        n53 = global write "Global Settings.vi" "Arrow Color"("Robot Color") -> ()
        n54 = Unbundle(w142) -> ("width"=w141:dbl, "height"=w140:dbl, w137:dbl, w136:dbl)
        n55 = Bundle("width"=w141, "height"=w140) -> (w139:cluster{"width":dbl, "height":dbl})  [unwired: 1 in]
        n56 = Bundle(w136, w137) -> (w138:cluster{dbl, dbl})  [unwired: 1 in]
        n57 = property on="Picture" class="Pict"("Position"=w139) -> ()  [unwired: 2 in, 2 out]
        n58 = property on="Picture" class="Pict"("Draw Area Size"=w138) -> ()  [unwired: 2 in, 2 out]
        n59 = First Call?() -> (First Call?: T/F=w163:bool)
      }
      event "Push": Value Change {
        # "Times out after\n5s"
        n60 = event-data() -> ()  [unwired: 1 in, 6 out]
        n61 = call <vilib>:"Set Busy.vi"() -> ("error out"=w185:errorcluster)  [unwired: 10 in, 1 out]
        n62 = local read "Open"() -> (w201:i32[])
        n63 = property on="Open" class="MCListbox (strict)"(error in=w185) -> ("ItemNames"=w200:string[][])  [unwired: 1 in, 2 out]
        n64 = Array Size(array=w201) -> (size(s)=w202:i32)
        n65 = Index Array(array=w201) -> (element=w203:i32)  [unwired: 1 in]
        n66 = Unbundle(w209) -> ("Updated Waypoints"=w208:cluster{"x":dbl, "y":dbl, "th":dbl}[])  [unwired: 3 out]
        n67 = Array Subset(array=w200, index (row)=w203, length (row)=w202) -> (w199:string[][])  [unwired: 2 in]
        n68 = for {
          tunnel: w199 -> [w239] mode=indexing
          tunnel: w206 -> [w233]
          tunnel: [w234] -> w198 mode=indexing
          n69 = Index Array(array=w239, index=0) -> (element=w232:string)
          n70 = Build Path(base path=w233, name or relative path=w232) -> (appended path=w231:path)
          n71 = Concatenate Strings("/home/lvuser/natinst/bin/Paths/" ("string"), w232) -> (w236:string)
          n72 = Bundle(w236, "appended path"=w231, TRUE) -> (w234:cluster{string, "appended path":path, bool})  [unwired: 1 in]
        }
        n73 = String To IP() -> (0:w192:u32)  [unwired: 1 in]
        n74 = IP To String(1:TRUE ("dot notation? (F)"), 2:w192) -> (0:w186:string)
        n75 = String Subset(string=w186, length (rest)=9 ("length (rest)")) -> (substring=w189:string)  [unwired: 1 in]
        n76 = Concatenate Strings(w189, "2" ("string")) -> (w187:string)
        n77 = call "Put Multiple Files.vi"("active (T)"=FALSE, "password"="", "user"="anonymous", "Open Connection Timeout (ms)"=5000.0, "file specifications"=w198, "host"=w187) -> ("error out"=w194:errorcluster, "file errors"=w195:errorcluster[])  [unwired: 4 in]
        n78 = Merge Errors(w195, w194) -> (w193:errorcluster)
        n79 = case shown="Error .." w193 {
          selector: w193 -> [_ w218]
          tunnel: [w214 w215] -> w184
          frame No Error {
            n80 = call "Successful"() -> ("error out"=w214:errorcluster)  [unwired: 10 in, 1 out]
          }
          frame Error {
            n81 = Equal?(x=w218, y=errorcluster {"status"=TRUE, "code"=56, "source"=""}) -> (x = y?=w222:T24)
            n82 = Unbundle By Name(w222) -> ("status"=w221:bool, "code"=w220:bool)
            n83 = Unbundle By Name(w218) -> ("code"=w216:i32, "source"=w217:string)
            n84 = And(x=w221, y=w220) -> (x .and. y?=w219:bool)
            n85 = case shown="True" w219 {
              tunnel: w217 -> [w228 _]
              tunnel: w216 -> [w227 _]
              tunnel: [w224 w230] -> w215
              frame False {
                n86 = Number To Decimal String(number=w227) -> (decimal integer string=w226:string)  [unwired: 1 in]
                n87 = Concatenate Strings("Error pushing the paths. Please see below for details:\n" ("string"), w228, w226) -> (w225:string)
                n88 = call "Error"("Message"=w225) -> ("error out"=w224:errorcluster)  [unwired: 9 in, 1 out]
              }
              frame True {
                n89 = call "Error"() -> ("error out"=w230:errorcluster)  [unwired: 10 in, 1 out]
              }
            }
          }
        }
        n90 = call <vilib>:"Unset Busy.vi"("error in (no error)"=w184) -> ()  [unwired: 10 in, 1 out]
      }
      event "New": Value Change {
        w240 = TRUE
        # "Button was pushed. Create a new trajectory path"
        # "Use Initial Location"
        n91 = event-data() -> ()  [unwired: 1 in, 5 out]
        n92 = Unbundle(w247) -> ("Updated Waypoints"=w246:cluster{"x":dbl, "y":dbl, "th":dbl}[])  [unwired: 3 out]
        n93 = local write "Conditions"(T10 {"vInitial (fps)"=0.0, "vFinal (fps)"=0.0} ("Conditions")) -> ()
      }
      event "Append": Value Change {
        # "Append button was pressed. Create a trajectory file that adopts the current position, heading, and start velocity"
        n94 = event-data() -> ()  [unwired: 1 in, 1 out]
        n95 = Unbundle(w269) -> ("Updated Waypoints"=w250:cluster{"x":dbl, "y":dbl, "th":dbl}[])  [unwired: 3 out]
        n96 = Array Size(array=w250) -> (size(s)=w259:i32)
        n97 = Decrement(x=w259) -> (x-1=w257:i32)
        n98 = Decrement(x=w257) -> (x-1=w258:i32)
        n99 = Index Array(array=w250, index=w257) -> (element=w262:cluster{"x":dbl, "y":dbl, "th":dbl})
        n100 = Index Array(array=w250, index=w258) -> (element=w256:cluster{"x":dbl, "y":dbl, "th":dbl})
        n101 = Unbundle(w262) -> ("x"=w255:dbl, "y"=w254:dbl, "th"=w261:dbl)
        n102 = Unbundle(w256) -> ("x"=w253:dbl, "y"=w252:dbl)  [unwired: 1 out]
        n103 = Not A Number/Path/Refnum?(number/path/refnum=w261) -> (NaN/Path/Refnum?=w260:bool)
        n104 = case shown="True" w260 {
          tunnel: w255 -> [_ w293]
          tunnel: w254 -> [_ w292]
          tunnel: w253 -> [_ w295]
          tunnel: w252 -> [_ w294]
          tunnel: [w283 w289] -> w251
          tunnel: w250 -> [w283 w291]
          frame False {
          }
          frame True {
            n105 = Subtract(x=w293, y=w295) -> (x-y=w284:dbl)
            n106 = Subtract(x=w292, y=w294) -> (x-y=w285:dbl)
            n107 = Delete From Array(array=w291) -> (array with subset deleted=w290:cluster{"x":dbl, "y":dbl, "th":dbl}[])  [unwired: 2 in, 1 out]
            n108 = Inverse Tangent (2 Input)(1:w284, 2:w285) -> (0:w288:dbl)
            n109 = expression code="(x/pi)*180.0" "radians to degrees"(w288) -> (w287:dbl)
            n110 = Bundle("x"=w293, "y"=w292, w287) -> (w286:cluster{"x":dbl, "y":dbl, dbl})  [unwired: 1 in]
            n111 = Build Array (concatenate)(w290, w286) -> (w289:cluster{"x":dbl, "y":dbl, "th":dbl}[])
          }
        }
        n112 = local read "Conditions"() -> (w278:T10)
        n113 = local read "Limits"() -> (w274:T9)
        n114 = Unbundle(w274) -> ("Velocity (fps)"=w273:dbl, "Accel (fps^2)"=w272:dbl)  [unwired: 2 out]
        n115 = Delete From Array(array=w251) -> (deleted portion=w280:cluster{"x":dbl, "y":dbl, "th":dbl})  [unwired: 2 in, 1 out]
        n116 = Divide(x=w273, y=w272) -> (x/y=w282:dbl)
        n117 = Build Array(w280) -> (w279:cluster{"x":dbl, "y":dbl, "th":dbl}[])
        n118 = Unbundle(w278) -> ("vFinal (fps)"=w277:dbl)  [unwired: 1 out]
        n119 = call "Add First Point.vi"("Accel (f/s^2)"=w272, "Time (s)"=w282, "Initial Points"=w279) -> ("Points"=w281:cluster{"x":dbl, "y":dbl, "th":dbl}[])  [unwired: 8 in]
        n120 = Bundle("vFinal (fps)"=w277, 0.0) -> (w276:cluster{"vFinal (fps)":dbl, dbl})  [unwired: 1 in]
        n121 = local write "Conditions"(w276) -> ()
      }
      event "Play": Value Change {
        # "Play button was pressed. Start playing the path by firing the event where it will self-feed."
        n122 = event-data() -> ()  [unwired: 1 in, 1 out]
        n123 = Unbundle(w301) -> ("Updated Waypoints"=w300:cluster{"x":dbl, "y":dbl, "th":dbl}[])  [unwired: 3 out]
        n124 = Tick Count (ms)() -> (millisecond timer value=w302:u32)
        n125 = Generate User Event(user event=w304, event data cluster=w302) -> ()  [unwired: 2 in, 2 out]
      }
      event "Save": Value Change {
        # "Negate timeout to immed update list of files"
        # "Save button was pressed. Save the file to the current directory.\nIf you modify the save code, be sure to update load as well."
        n126 = event-data() -> ()  [unwired: 1 in, 1 out]
        n127 = Unbundle By Name(w322) -> ("Time (s)"=w315:dbl, "Distance (ft)"=w320:dbl)
        n128 = Unbundle(w338) -> ("Trajectory Data"=w329:T12, "Updated Waypoints"=w330:cluster{"x":dbl, "y":dbl, "th":dbl}[], w328:T14)  [unwired: 1 out]
        n129 = local read "Drive Type"() -> (w325:T11)
        n130 = local read "Path Type"() -> (w324:T7)
        n131 = for {
          tunnel: w316 -> [w350] mode=indexing
          tunnel: w315 -> [w349]
          shift-right: [w345] -> w311
          shift-left: "" -> [w347]
          n132 = Unbundle(w350) -> ("Time (s)"=w343:dbl, w348:T3)  [unwired: 1 out]
          n133 = Unbundle By Name(w348) -> ("Name"=w344:string)
          n134 = Greater?(x=w343, y=w349) -> (0:w346:bool)
          n135 = case shown="True" w346 {
            tunnel: w347 -> [w351 w359]
            tunnel: [w351 w358] -> w345
            tunnel: w344 -> [_ w355]
            tunnel: w343 -> [_ w357]
            frame False {
            }
            frame True {
              n136 = Format Value(format string="%.2f", value (0)=w357) -> (output string=w353:string)  [unwired: 1 in]
              n137 = Concatenate Strings(w359, w355, " at " ("string"), w353, " seconds \n" ("string")) -> (w358:string)
            }
          }
        }
        n138 = Bundle("Drive Type"=w325, "Path Type"=w324) -> (w323:cluster{"Drive Type":T11, "Path Type":T7})  [unwired: 1 in]
        n139 = Select(t=nan, s="Zero Velocity", f=w320) -> (s? t:f=w318:dbl)
        n140 = Bundle("Time (s)"=w315, "Distance (ft)"=w318) -> (w317:cluster{"Time (s)":dbl, "Distance (ft)":dbl})  [unwired: 1 in]
        n141 = String Length(string=w311) -> (length=w313:i32)
        n142 = Bundle("Robot Backwards"="Robot Backwards", "Reverse Path"="Reverse Path") -> (w331:T25)  [unwired: 1 in]
        n143 = Not Equal To 0?(x=w313) -> (x != 0?=w312:bool)
        n144 = case shown="True" w312 {
          tunnel: w311 -> [_ w341]
          frame False {
          }
          frame True {
            n145 = Concatenate Strings("You have command(s) that will not be executed during this path.\nThese include:\n", w341) -> (w340:string)
            n146 = call "Display Message to User"("Message"=w340) -> ()  [unwired: 9 in, 2 out]
          }
        }
        n147 = Bundle(w331, "Trajectory Data"=w329, "sorted array out"=w316, w328, "Updated Waypoints"=w330, w317, "Zero Velocity"="Zero Velocity", w323, "Pickup Balls"="Pickup Balls", "Current Limit"="Current Limit", "Zero Translational\n Velocity"="Zero Translational\n Velocity", "Correct at Beginning \nof Path"="Correct at Beginning \nof Path") -> (w308:T26)  [unwired: 1 in]